vi "RAKE(4800).vi"(0 "Номер\nканала":i32, 7 "add":bool, 11 "ВЫБОРКА":cdb format="%#.6g") -> ()   [LabVIEW 2013]
uses:
  common/Viterbi.vi
  FER(4800).vi
  common/metrics.vi
  transmitter/4800/syndrom(4800).vi
  Gateway(4800).vi
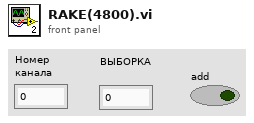
[diagram p1: front panel]
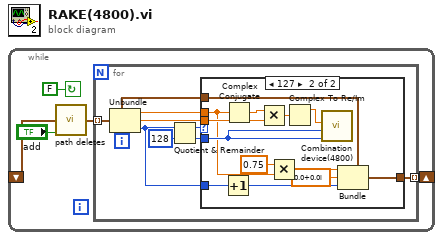
[diagram p0: block diagram]
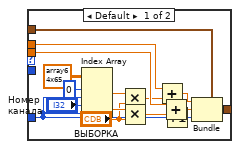
[diagram p2: hidden frame]
diagram:
  n1 = while {
    shift-right: [w2] -> _
    shift-left: _ -> [w3]
    stop <- FALSE continue-if-true
    n2 = call "path deletes.vi"("paths in"=w3, "new path"="add") -> ("path out"=w4:cluster{cdb, cdb, i32}[])  [unwired: 13 in]
    n3 = for {
      tunnel: [w10] -> w2 mode=indexing
      tunnel: w4 -> [w6] mode=indexing
      n4 = Unbundle(w6) -> (w11:cdb, w12:cdb, w9:i32)
      n5 = Quotient & Remainder(x=w9, y=128) -> (x-y*floor(x/y)=w8:i32, floor(x/y)=w7:i32)
      n6 = case shown="127" w8 {
        tunnel: w9 -> [w22 w41]
        tunnel: w12 -> [w24 w40]
        tunnel: w11 -> [w18 w31]
        tunnel: [w23 w38] -> w10
        tunnel: w7 -> [_ w35]
        tunnel: w6 -> [w14 w30]
        frame Default {
          n7 = Index Array(array=cdb[][] array64x65536[4194304 elements] ("Modificated signals 2"), index (row) #1=0, index (col) #1=w22, index (row) #2="Номер\nканала", index (col) #2=w22) -> (element #1=w17:cdb, element #2=w26:cdb)
          n8 = Multiply(x=w17, y="ВЫБОРКА") -> (x*y=w20:cdb)
          n9 = Multiply(x=w26, y="ВЫБОРКА") -> (x*y=w29:cdb)
          n10 = Add(x=w18, y=w20) -> (x+y=w19:cdb)
          n11 = Add(x=w24, y=w29) -> (x+y=w25:cdb)
          n12 = Increment(x=w22) -> (x+1=w28:i32)
          n13 = Bundle(cluster=w14, w19, w25, w28) -> (w23:cluster{cdb, cdb, i32})
        }
        frame 127 {
          n14 = Increment(x=w41) -> (x+1=w37:i32)
          n15 = Complex Conjugate(1:w31) -> (0:w32:cdb)
          n16 = Multiply(x=w32, y=w40) -> (x*y=w42:cdb)
          n17 = Multiply(x=0.75, y=w31) -> (x*y=w34:cdb)
          n18 = Complex To Re/Im(x + iy=w42) -> (x=w36:dbl)  [unwired: 1 out]
          n19 = call "Combination device(4800).vi"("i"=w35, "Фаза 2"=w35, "Значение пика"=w36) -> ()  [unwired: 9 in]
          n20 = Bundle(cluster=w30, w34, cdb 0.0+0.0i, w37) -> (w38:cluster{cdb, cdb, i32})
        }
      }
    }
  }
